vi "UHR-Fleezers Control (host) - 10.8MV_trial.vi"() -> ()   [LabVIEW 2010] (continued)
        n689 = local read "X RF Frequency Limits (MHz)"() -> (w3468:T16)
        n690 = local read "Y RF Frequency Limits (MHz)"() -> (w3465:T16)
        n691 = local read "BD 2 Frequency 1 (MHz)"() -> (w3470:dbl)
        n692 = Negate(x="Scan Range (nm)") -> (-x=w3434:dbl)
        n693 = Divide(x=w3434, y=w3456) -> (x/y=w3438:dbl)
        n694 = Select(t=w3468, s="Scan BD", f=w3465) -> (s? t:f=w3467:T16)
        n695 = Select(t=w3464, s="Scan BD", f=w3470) -> (s? t:f=w3469:dbl)
        n696 = Unbundle By Name(w3467) -> ("Maximum"=w3476:dbl, "Minimum"=w3475:dbl)
        n697 = Add(x=w3438, y=w3469) -> (x+y=w3473:dbl)
        n698 = Divide(x=w3434, y="Step Size (nm)") -> (x/y=w3453:dbl)
        n699 = Divide(x="Step Size (nm)", y=w3456) -> (x/y=w3462:dbl)
        n700 = Absolute Value(x=w3453) -> (abs(x)=w3437:dbl)
        n701 = Sign(1:w3434) -> (0:w3435:dbl)
        n702 = In Range and Coerce(upper limit=w3476, x=w3473, lower limit=w3475) -> (coerced(x)=w3472:dbl, In Range?=w3474:bool)
        n703 = To Unsigned Quad Integer(1:w3437) -> (0:w3452:u64)
        "Scan steps (AOD)" <- w3452
        n704 = call "IR AOM freq to word.vi"("Frequency In (MHz)"=w3462) -> ("Frequency Word Out (double)"=w3459:dbl)
        n705 = Multiply(x=w3435, y=w3459) -> (x*y=w3436:dbl)
        n706 = Subtract(x=w3473, y=w3472) -> (x-y=w3471:dbl)
        n707 = To Quad Integer(1:w3436) -> (0:w3458:i64)
        "Incr. int (AOD)" <- w3458
        n708 = Subtract(x=w3438, y=w3471) -> (x-y=w3457:dbl)
        "Scan Range (MHz)" <- w3457
        n709 = Select(t=w3438, s=w3474, f=w3457) -> (s? t:f=w3477:dbl)
        n710 = Multiply(x=w3457, y=w3456) -> (x*y=w3455:dbl)
        n711 = Decrement(x=w3452) -> (x-1=w3505:u64)
        n712 = Negate(x=w3455) -> (-x=w3451:dbl)
        n713 = local write "Scan Range (nm)"(w3451) -> ()
        n714 = Divide(x=w3477, y=w3505) -> (x/y=w3461:dbl)
        "Scan Increment (MHz)" <- w3461
        n715 = call "IR AOM freq to word.vi"("Frequency In (MHz)"=w3461) -> ("Frequency Word Out (double)"=w3460:dbl)
        n716 = Divide(x="Step Size (nm)", y="Scan Speed (nm/s)") -> (x/y=w3448:dbl)
        n717 = To Quad Integer(1:w3460) -> ()  [unwired: 1 out]
        n718 = local read "Number Interlace Sets"() -> (w3432:u8)
        n719 = local read "AI Count (ticks)"() -> (w3433:u32)
        n720 = local read "Total Counts (ticks)"() -> (w3431:u32)
        n721 = local read "# Samples/trap"() -> (w3463:u32)
        n722 = Multiply(x=w3433, y=w3432) -> (x*y=w3430:u32)
        n723 = Divide(x=w3431, y=w3430) -> (x/y=w3429:dbl)
        n724 = Select(t=w3464, s="Scan BD", f=w3470) -> (s? t:f=w3502:dbl)
        "Initial freq. (MHz)" <- w3502
        n725 = Add(x=w3477, y=w3502) -> (x+y=→"Final freq. (MHz)":dbl)
        n726 = Divide(x=w3431, y=40000000.0) -> (x/y=w3447:dbl)
        n727 = Divide(x=w3448, y=w3447) -> (x/y=w3446:dbl)
        n728 = To Unsigned Quad Integer(1:w3446) -> (0:w3421:u64)
        n729 = Quotient & Remainder(x=w3421, y=u64 2) -> (x-y*floor(x/y)=w3425:u64)  [unwired: 1 out]
        n730 = Equal?(x=w3425, y=u64 0) -> (x = y?=w3423:bool)
        n731 = Decrement(x=w3421) -> (x-1=w3422:u64)
        n732 = Select(t=w3421, s=w3423, f=w3422) -> (s? t:f=w3420:u64)
        "Cycles/step (AOD)" <- w3420
        n733 = xnode "Read/Write Control"("FPGA VI Reference In"=w3513, "error in"=w3512, "Scan steps"=w3452, "Number of scans"="Number of F/B Scans (AOD)", "Cycles per step"=w3420, "Scan freq.  increment"=w3458, "Scan BD"="Scan BD") -> ("error out"=w3511:errorcluster)  [unwired: 1 out]
        n734 = Multiply(x=w3452, y=w3420) -> (x*y=w3506:u64)
        n735 = Multiply(x=w3506, y=u64 2) -> (x*y=w3428:u64)
        n736 = Multiply(x=w3429, y=w3428) -> (x*y=w3427:dbl)
        "Data points/scan (f/b)" <- w3427
        n737 = Multiply(x=w3427, y="Number of F/B Scans (AOD)") -> (x*y=w3509:dbl)
        "Data points/scans" <- w3509
        n738 = Divide(x=w3509, y=w3463) -> (x/y=→"N sets should be saved":dbl)
        n739 = Multiply(x=w3506, y=w3447) -> (x*y=w3445:dbl)
        "Time/Scan (s) (AOD)" <- w3445
        n740 = Select(t=w3477, s="Scan BD", f=0.0) -> (s? t:f=w3503:dbl)
        n741 = Select(t=0.0, s="Scan BD", f=w3477) -> (s? t:f=w3499:dbl)
        n742 = local read "BD 2 Frequency 2 (MHz)"() -> (w3495:dbl)
        n743 = local read "BD 1 Frequency 2 (MHz)"() -> (w3498:dbl)
        n744 = Add(x=w3499, y=w3470) -> (x+y=w3496:dbl)
        n745 = Add(x=w3464, y=w3503) -> (x+y=w3497:dbl)
        n746 = Multiply(x=w3445, y=2.0) -> (x*y=w3444:dbl)
        n747 = Multiply(x=w3444, y="Number of F/B Scans (AOD)") -> (x*y=w3441:dbl)
        n748 = Divide(x=w3441, y=60.0) -> (x/y=→"Time to Finish All (min)":dbl)
        n749 = Add(x="Trap 2 Bead Size (nm)", y="Trap 1 Bead Size (nm)") -> (x+y=w3485:dbl)
        n750 = local read "Initial delta (MHz)"() -> (w3482:dbl)
        n751 = Divide(x=w3485, y=2.0) -> (x/y=w3479:dbl)
        n752 = Subtract(x=w3496, y=w3495) -> (x-y=w3493:dbl)
        n753 = Subtract(x=w3497, y=w3498) -> (x-y=w3494:dbl)
        n754 = Square(x=w3493) -> (x^2=w3492:dbl)
        n755 = Square(x=w3494) -> (x^2=w3491:dbl)
        n756 = Add(x=w3491, y=w3492) -> (x+y=w3490:dbl)
        n757 = Square Root(x=w3490) -> (sqrt(x)=w3489:dbl)
        "Final delta (MHz)" <- w3489
        n758 = Multiply(x=w3481, y=w3489) -> (x*y=w3488:dbl)
        n759 = Multiply(x=w3482, y=w3481) -> (x*y=w3480:dbl)
        n760 = Subtract(x=w3480, y=w3479) -> (x-y=→"Initial sep (nm)":dbl)
        n761 = Subtract(x=w3488, y=w3479) -> (x-y=→"Final sep (nm)":dbl)
      }
      event "Raster Scanning...": Value Change {
        n762 = event-data() -> ("NewVal"=w3650:bool)  [unwired: 6 out]
        n763 = case shown="True" w3650 {
          frame False {
          }
          frame True {
            n764 = property on="BD 1 Frequency 1 (MHz)" class="DigNum (strict)"("Val(Sgnl)"=65.0 ("Value (Signaling)")) -> ()  [unwired: 2 in, 2 out]
          }
        }
      }
      event "Freq or Amp switch first", "Swap F1 and F2", "Freq switch delay", "Amp switch delay": Value Change {
        n765 = event-data() -> ()  [unwired: 7 out]
        n766 = local read "Freq or Amp switch first"() -> (w3652:bool)
        n767 = local read "Amp switch delay"() -> (w3653:u16)
        n768 = local read "Freq switch delay"() -> (w3655:u16)
        n769 = local read "Swap F1 and F2"() -> (w3654:bool)
        n770 = xnode "Read/Write Control"("FPGA VI Reference In"=w3658, "error in"=w3657, "Freq switch delay"=w3655, "Swap F1 and F2"=w3654, "Amp switch delay"=w3653, "Freq or Amp switch first"=w3652) -> ("error out"=w3656:errorcluster)  [unwired: 1 out]
      }
      event "Scan steps (MCL)", "Number of scans (MCL)", "Scan Range (V)\n(of steps)", "2D or 1D Scan", "N APD Samp/step", "Fast Scan Dir", "Continuous MCL Scanning", "Scan lines (y)": Value Change {
        w3759 = 32767.0 ("y")
        n771 = event-data() -> ()  [unwired: 7 out]
        n772 = Select(t="Scan lines (y)", s="2D or 1D Scan", f="Number of scans (MCL)") -> (s? t:f=w3764:u64)
        n773 = Decrement(x="Scan steps (MCL)") -> (x-1=w3780:u64)
        n774 = Divide(x="Scan Range (V)\n(of steps)", y=w3780) -> (x/y=w3779:dbl)
        "Desired Scan Incr (V)" <- w3779
        n775 = local read "APD Integration Time (s)"() -> (w3772:dbl)
        n776 = Multiply(x=w3779, y=w3759) -> (x*y=w3788:dbl)
        n777 = Divide(x=w3788, y=10.0) -> (x/y=w3778:dbl)
        "Desired incr (int)" <- w3778
        n778 = local read "Update Count (MCL)"() -> (w3784:u32)
        n779 = Round Toward -Infinity(1:w3778) -> (0:w3787:dbl)
        n780 = To Word Integer(number=w3787) -> (16bit integer=w3762:i16)
        "Actual Incr. int (MCL)" <- w3762
        n781 = Multiply(x=w3772, y=40000000.0) -> (x*y=w3785:dbl)
        n782 = Divide(x=w3785, y=w3784) -> (x/y=w3783:dbl)
        n783 = Multiply(x=i16 10, y=w3762) -> (x*y=w3760:i16)
        n784 = Multiply(x="N APD Samp/step", y=w3783) -> (x*y=w3782:dbl)
        "Cycles/step (MCL)" <- w3782
        n785 = Divide(x=w3760, y=w3759) -> (x/y=→"Actual MCL Inc (V)":dbl)
        n786 = Multiply(x="N APD Samp/step", y="Scan steps (MCL)") -> (x*y=w3774:dbl)
        n787 = local read "APD Samples/FIFO Acq."() -> (w3771:dbl)
        n788 = Multiply(x=w3774, y=u64 2) -> (x*y=w3773:dbl)
        "Data points/scan (f+b)" <- w3773
        n789 = Multiply(x=w3773, y=w3764) -> (x*y=w3791:dbl)
        "Data points/scans (MCL)" <- w3791
        n790 = Multiply(x=w3772, y=w3773) -> (x*y=w3765:dbl)
        "Time/f+b scan (s) (MCL)" <- w3765
        n791 = Divide(x=w3791, y=w3771) -> (x/y=→"N sets should be saved (MCL)":dbl)
        n792 = Multiply(x=w3765, y=w3764) -> (x*y=→"Total Time (s)":dbl)
        n793 = Not(x="Fast Scan Dir") -> (.not. x?=w3769:bool)
        n794 = xnode "Read/Write Control"("FPGA VI Reference In"=w3795, "error in"=w3794, "Scan steps (MCL)"="Scan steps (MCL)", "Number of scans (MCL)"=w3764, "Cycles per step (MCL)"=w3782, "Scan freq.  increment (MCL)"=w3762, "1D or 2D Scan?"="2D or 1D Scan", "MCL Scan Axis"=w3769, "Cont. Scan (MCL)"="Continuous MCL Scanning") -> ("error out"=w3793:errorcluster)  [unwired: 1 out]
      }
      event "Read Cal": Value Change {
        w3969 = 1000.0 ("y")
        n795 = event-data() -> ()  [unwired: 7 out]
        n796 = local read "Save file name"() -> (w3994:path)
        n797 = local write "Read Cal"(FALSE ("Read Cal")) -> ()
        n798 = Strip Path(path=w3994) -> (stripped path=w3993:path)  [unwired: 1 out]
        n799 = Path To String(path=w3993) -> (string=w3992:string)
        n800 = Concatenate Strings(w3992, "\\current.cal" ("string")) -> (w3990:string)
        n801 = String To Path(string=w3990) -> (path=w3989:path)
        n802 = Open/Create/Replace File(file path (use dialog)=w3989, operation (0:open)=T25."open", access (0:read/write)=enum16{"read/write", "read-only", "write-only"}."read-only") -> (refnum out=w3997:refnum<file>, error out=w3983:errorcluster)  [unwired: 1 in, 3 out]
        n803 = Deny Access(4:w3983, 7:w3997) -> (0:w3982:errorcluster, 3:w3988:refnum<file>)  [unwired: 1 out]
        n804 = Read from Binary File(5:0.0, 8:w3982, 9:T31."big-endian, network order" ("byte order (0:big-endian, network order)"), 10:-1 ("count (1)"), 11:w3988) -> (0:w3981:errorcluster, 2:w3979:dbl[], 3:w3984:refnum<file>)  [unwired: 2 out]
        n805 = Array To Cluster(array=w3979) -> (cluster=w3978:T33)
        n806 = Unbundle(w3978) -> ("[0]"=w3977:dbl, "[1]"=w3976:dbl, "[2]"=w3975:dbl, "[3]"=w3974:dbl, "[4]"=w3973:dbl, "[5]"=w3972:dbl)
        n807 = Close File(refnum=w3984, error in=w3981) -> (error out=→"Read cal error":errorcluster)  [unwired: 1 out]
        n808 = Multiply(x=w3972, y=w3969) -> (x*y=w3970:dbl)
        n809 = local write "T2 kappa_x (pN/nm)"(w3974) -> ()
        n810 = local write "T1 kappa_x (pN/nm)"(w3975) -> ()
        n811 = local write "T1 alpha_x (nm/V)"(w3977) -> ()
        n812 = local write "T2 alpha_x (nm/V)"(w3976) -> ()
        n813 = Multiply(x=w3973, y=w3969) -> (x*y=w3971:dbl)
        n814 = local write "T1 offset_x (mV)"(w3971) -> ()
        n815 = local write "T2 offset_x (mV)"(w3970) -> ()
      }
      event "Abort MCL Scan": Value Change {
        n816 = event-data() -> ()  [unwired: 7 out]
        n817 = local write "MCL Scanning"(FALSE ("MCL Scanning")) -> ()
        n818 = xnode "Read/Write Control"("FPGA VI Reference In"=w4002, "error in"=w4001, "Abort scan (MCL)"="Abort MCL Scan") -> ("error out"=w4000:errorcluster)  [unwired: 1 out]
      }
      event "Update Count (MCL)": Value Change {
        n819 = event-data() -> ()  [unwired: 7 out]
        n820 = xnode "Read/Write Control"("FPGA VI Reference In"=w4044, "error in"=w4043, "MCL count"="Update Count (MCL)") -> ("error out"=w4042:errorcluster)  [unwired: 1 out]
      }
      event "Phase adjust (MCL)", "+ phase (MCL)", "- phase (MCL)": Value Change {
        n821 = event-data() -> ()  [unwired: 7 out]
        n822 = Negate(x="Phase adjust (MCL)") -> (-x=w4090:i16)
        n823 = Select(t=w4090, s="- phase (MCL)", f="Phase adjust (MCL)") -> (s? t:f=w4088:i16)
        n824 = Or(x="- phase (MCL)", y="+ phase (MCL)") -> (x .or. y?=w4083:bool)
        n825 = xnode "Read/Write Control"("FPGA VI Reference In"=w4092, "error in"=w4091, "Phase count adjustment (MCL)"=w4088) -> ("FPGA VI Reference Out"=w4084:T19, "error out"=w4085:errorcluster)
        n826 = xnode "Read/Write Control"("FPGA VI Reference In"=w4084, "error in"=w4085, "+ phase (MCL)"=w4083) -> ("error out"=w4082:errorcluster)  [unwired: 1 out]
      }
      event "Abort AOD Scan": Value Change {
        n827 = event-data() -> ()  [unwired: 7 out]
        n828 = xnode "Read/Write Control"("FPGA VI Reference In"=w4171, "error in"=w4170, "Abort scan"="Abort AOD Scan") -> ("error out"=w4169:errorcluster)  [unwired: 1 out]
      }
      event "Continuous AOD Scanning": Value Change {
        n829 = event-data() -> ()  [unwired: 7 out]
        n830 = xnode "Read/Write Control"("FPGA VI Reference In"=w4213, "error in"=w4212, "Cont. Scan"="Continuous AOD Scanning") -> ("error out"=w4211:errorcluster)  [unwired: 1 out]
      }
      event "Index": Value Change {
        n831 = event-data() -> ()  [unwired: 7 out]
        n832 = call "Create new save file.vi"("Insert"="", "Ext"=".dat" ("string"), "Index In"="Index") -> ("Path Out"=→"Save file name":path, "Index Out"=w4252:dbl)
        "Save index" <- w4252
        n833 = local write "Index"(w4252) -> ()
      }
      event "AO1", "AO2": Value Change {
        w4267 = 10.0 ("y")
        w4266 = 32767.0 ("y")
        n834 = event-data() -> ()  [unwired: 7 out]
        n835 = local read "AO2"() -> (w4265:dbl)
        n836 = local read "AO1"() -> (w4262:dbl)
        n837 = Multiply(x=w4262, y=w4266) -> (x*y=w4261:dbl)
        n838 = Multiply(x=w4265, y=w4266) -> (x*y=w4264:dbl)
        n839 = Divide(x=w4261, y=w4267) -> (x/y=w4260:dbl)
        n840 = Divide(x=w4264, y=w4267) -> (x/y=w4263:dbl)
        n841 = To Word Integer(number=w4260) -> (16bit integer=w4268:i16)
        n842 = To Word Integer(number=w4263) -> (16bit integer=w4269:i16)
        n843 = xnode "Read/Write Control"("FPGA VI Reference In"=w4259, "error in"=w4258, "AO1"=w4268, "AO2"=w4269) -> ("error out"=w4257:errorcluster)  [unwired: 1 out]
      }
      event "Inject Bottom": Value Change {
        n844 = event-data() -> ()  [unwired: 7 out]
        n845 = disable-structure shown="Enabled" {
          disable-tunnel: "Inject Bottom" -> [w4328 w4368]
          frame Disabled {
            n846 = local read "Chemyx Syringe Pump Serial Port"() -> (w4329:refnum<visa-resource-name>)
            n847 = local read "Pump write delay (ms)"() -> (w4330:dbl)
            n848 = case shown="True" w4328 {
              tunnel: w4330 -> [w4336 w4350]
              tunnel: w4329 -> [w4333 w4349]
              frame False {
                n849 = flat-sequence {
                  tunnel: w4333 -> [w4337]
                  tunnel: [w4337] -> w4334
                  tunnel: w4336 -> [_]
                  tunnel: [w4340] -> w4335
                  tunnel: w4334 -> [w4340]
                  tunnel: w4335 -> [w4341]
                  tunnel: [w4341] -> w4331
                  tunnel: [w4343] -> w4332
                  tunnel: w4331 -> [w4343]
                  tunnel: w4332 -> [w4345]
                  frame #0 {
                    n850 = call "Write to pump.vi"("string"="enter pump1", "VISA resource name"=w4337) -> ()  [unwired: 1 out]
                  }
                  frame #1 {
                    n851 = Wait (ms)(milliseconds to wait="Pump pause delay (ms)") -> ()  [unwired: 1 out]
                  }
                  frame #2 {
                    n852 = call "Write to pump.vi"("string"="stop", "VISA resource name"=w4341) -> ()  [unwired: 1 out]
                  }
                  frame #3 {
                    n853 = Wait (ms)(milliseconds to wait=u32 500) -> ()  [unwired: 1 out]
                  }
                  frame #4 {
                    n854 = call "Write to pump.vi"("string"="stop", "VISA resource name"=w4345) -> ()  [unwired: 1 out]
                  }
                }
              }
              frame True {
                n855 = flat-sequence {
                  tunnel: w4349 -> [w4359]
                  tunnel: w4350 -> [w4354]
                  tunnel: w4350 -> [w4361]
                  tunnel: w4349 -> [w4362]
                  tunnel: [w4362] -> w4347
                  tunnel: [w4364] -> w4348
                  tunnel: w4347 -> [w4364]
                  tunnel: w4348 -> [w4366]
                  frame #0 {
                    n856 = local read "All Pump Parameters"() -> (w4353:T5)
                    n857 = Unbundle By Name(w4353) -> ("Pump 1"=w4360:T34)
                    n858 = call "Set pump parameters.vi"("Pump write delay (ms)"=w4354, "Volume (uL)"="Ch 2 Inject Volume (uL)", "Rate (uL/h)"="Ch 1 Inject Rate (ul/h)", "Units"=4.0, "Pump #"=1.0, "Pump Parameters In"=w4360, "VISA resource name"=w4359) -> ("Pump Parameters Out"=w4352:T34)  [unwired: 3 in]
                    n859 = Bundle By Name(cluster=w4353, "Pump 1"=w4352) -> (w4351:T5)
                    n860 = local write "All Pump Parameters"(w4351) -> ()
                  }
                  frame #1 {
                    n861 = Wait (ms)(milliseconds to wait=w4361) -> ()  [unwired: 1 out]
                  }
                  frame #2 {
                    n862 = call "Write to pump.vi"("string"="start", "VISA resource name"=w4362) -> ()  [unwired: 1 out]
                  }
                  frame #3 {
                    n863 = Wait (ms)(milliseconds to wait=u32 500) -> ()  [unwired: 1 out]
                  }
                  frame #4 {
                    n864 = call "Write to pump.vi"("string"="start", "VISA resource name"=w4366) -> ()  [unwired: 1 out]
                  }
                }
              }
            }
          }
          frame Enabled {
            n865 = call "hamilton_controller.vi"("Open?"=w4368, "valve"=enum16{"A", "B", "C", "D", "ALL"}."B", "action"=T22."MOVE VALVE") -> ()  [unwired: 8 in, 1 out]
          }
        }
      }
      event "Inject Top": Value Change {
        n866 = event-data() -> ()  [unwired: 7 out]
        n867 = disable-structure shown="Disabled" {
          disable-tunnel: "Inject Top" -> [_ w4412]
          frame Disabled {
            n868 = local read "Pump write delay (ms)"() -> (w4373:dbl)
            n869 = case shown="False" w4374 {
              tunnel: w4373 -> [w4380 w4394]
              tunnel: "Chemyx Syringe Pump Serial Port" -> [w4377 w4393]
              frame False {
                n870 = flat-sequence {
                  tunnel: w4377 -> [w4381]
                  tunnel: [w4381] -> w4378
                  tunnel: w4380 -> [_]
                  tunnel: [w4384] -> w4379
                  tunnel: w4378 -> [w4384]
                  tunnel: w4379 -> [w4385]
                  tunnel: [w4385] -> w4375
                  tunnel: [w4387] -> w4376
                  tunnel: w4375 -> [w4387]
                  tunnel: w4376 -> [w4389]
                  frame #0 {
                    n871 = call "Write to pump.vi"("string"="enter pump3", "VISA resource name"=w4381) -> ()  [unwired: 1 out]
                  }
                  frame #1 {
                    n872 = local read "Pump pause delay (ms)"() -> (w4383:u32)
                    n873 = Wait (ms)(milliseconds to wait=w4383) -> ()  [unwired: 1 out]
                  }
                  frame #2 {
                    n874 = call "Write to pump.vi"("string"="stop", "VISA resource name"=w4385) -> ()  [unwired: 1 out]
                  }
                  frame #3 {
                    n875 = Wait (ms)(milliseconds to wait=u32 0) -> ()  [unwired: 1 out]
                  }
                  frame #4 {
                    n876 = call "Write to pump.vi"("string"="stop", "VISA resource name"=w4389) -> ()  [unwired: 1 out]
                  }
                }
              }
              frame True {
                n877 = flat-sequence {
                  tunnel: w4393 -> [w4403]
                  tunnel: w4394 -> [w4398]
                  tunnel: w4394 -> [w4405]
                  tunnel: w4393 -> [w4406]
                  tunnel: [w4406] -> w4391
                  tunnel: [w4409] -> w4392
                  tunnel: w4391 -> [w4409]
                  tunnel: w4392 -> [w4410]
                  frame #0 {
                    n878 = local read "All Pump Parameters"() -> (w4397:T5)
                    n879 = Unbundle By Name(w4397) -> ("Pump 3"=w4404:T34)
                    n880 = call "Set pump parameters.vi"("Pump write delay (ms)"=w4398, "Volume (uL)"="Ch 3 Inject Volume (uL)", "Rate (uL/h)"="Ch 3 Inject Rate (ul/h)", "Units"=4.0, "Pump #"=3.0, "Pump Parameters In"=w4404, "VISA resource name"=w4403) -> ("Pump Parameters Out"=w4396:T34)  [unwired: 3 in]
                    n881 = Bundle By Name(cluster=w4397, "Pump 3"=w4396) -> (w4395:T5)
                    n882 = local write "All Pump Parameters"(w4395) -> ()
                  }
                  frame #1 {
                    n883 = Wait (ms)(milliseconds to wait=w4405) -> ()  [unwired: 1 out]
                  }
                  frame #2 {
                    n884 = call "Write to pump.vi"("string"="start", "VISA resource name"=w4406) -> ()  [unwired: 1 out]
                  }
                  frame #3 {
                    n885 = Wait (ms)(milliseconds to wait=u32 500) -> ()  [unwired: 1 out]
                  }
                  frame #4 {
                    n886 = call "Write to pump.vi"("string"="start", "VISA resource name"=w4410) -> ()  [unwired: 1 out]
                  }
                }
              }
            }
          }
          frame Enabled {
            n887 = call "hamilton_controller.vi"("Open?"=w4412, "valve"=enum16{"A", "B", "C", "D", "ALL"}."A", "action"=T22."MOVE VALVE") -> ()  [unwired: 8 in, 1 out]
          }
        }
      }
      event "Inject Valve B": Value Change {
        n888 = event-data() -> ()  [unwired: 7 out]
        n889 = disable-structure shown="Enabled" {
          disable-tunnel: "Inject Valve B" -> [w4416 w4436]
          frame Disabled {
            n890 = local read "Pump write delay (ms)"() -> (w4418:dbl)
            n891 = flat-sequence {
              tunnel: w4417 -> [w4431]
              tunnel: w4418 -> [w4427]
              tunnel: w4416 -> [_]
              tunnel: w4418 -> [w4433]
              tunnel: w4417 -> [w4434]
              frame #0 {
                n892 = local read "All Pump Parameters"() -> (w4426:T5)
                n893 = Multiply(x=60.0, y="Flush Center Ch Rate (ul/m)") -> (x*y=w4423:dbl)
                n894 = Unbundle By Name(w4426) -> ("Pump 2"=w4432:T34)
                n895 = call "Set pump parameters.vi"("Pump write delay (ms)"=w4427, "Volume (uL)"="Flush Center Ch Volume (uL)", "Rate (uL/h)"=w4423, "Units"=3.0, "Pump #"=2.0, "Pump Parameters In"=w4432, "VISA resource name"=w4431) -> ("Pump Parameters Out"=w4425:T34)  [unwired: 3 in]
                n896 = Bundle By Name(cluster=w4426, "Pump 2"=w4425) -> (w4424:T5)
                n897 = local write "All Pump Parameters"(w4424) -> ()
                n898 = Add(x="Flush Center Ch Volume (uL)", y="Total Volume\nFlushed (uL)") -> (x+y=w4420:dbl)
                n899 = local write "Total Volume\nFlushed (uL)"(w4420) -> ()
              }
              frame #1 {
                n900 = Wait (ms)(milliseconds to wait=w4433) -> ()  [unwired: 1 out]
              }
              frame #2 {
                n901 = call "Write to pump.vi"("string"="start", "VISA resource name"=w4434) -> ()  [unwired: 1 out]
              }
            }
            n902 = local read "Chemyx Syringe Pump Serial Port"() -> (w4417:refnum<visa-resource-name>)
          }
          frame Enabled {
            n903 = call "hamilton_controller.vi"("Open?"=w4436, "valve"=enum16{"A", "B", "C", "D", "ALL"}."B", "action"=T22."MOVE VALVE") -> ()  [unwired: 8 in, 1 out]
          }
        }
      }
      event "Sample Channel Flow": Value Change {
        n904 = event-data() -> ()  [unwired: 7 out]
        n905 = call "hamilton_controller.vi"("Open?"="Sample Channel Flow", "valve"=enum16{"A", "B", "C", "D", "ALL"}."C", "action"=T22."MOVE VALVE") -> ()  [unwired: 8 in, 1 out]
      }
      event "Flip Green Filter": Value Change {
        n906 = event-data() -> ()  [unwired: 7 out]
        n907 = Not(x="Flip Green Filter") -> (.not. x?=w4442:bool)
        n908 = local write "Flip Green Filter"(w4442) -> ()
        n909 = flat-sequence {
          tunnel: w4450 -> [w4455]
          tunnel: w4449 -> [w4454]
          tunnel: [w4452] -> w4447
          tunnel: [w4451] -> w4446
          tunnel: [w4495] -> w4445
          tunnel: w4447 -> [w4495]
          tunnel: [w4494] -> w4444
          tunnel: w4446 -> [w4494]
          tunnel: w4445 -> [w4499]
          tunnel: w4444 -> [w4498]
          tunnel: [w4497] -> w4448
          frame #0 {
            n910 = xnode "Read/Write Control"("FPGA VI Reference In"=w4455, "error in"=w4454, "Green Filter Flipper"=TRUE) -> ("FPGA VI Reference Out"=w4452:T19, "error out"=w4451:errorcluster)
          }
          frame #1 {
            n911 = Wait (ms)(milliseconds to wait=u32 100) -> ()  [unwired: 1 out]
          }
          frame #2 {
            n912 = xnode "Read/Write Control"("FPGA VI Reference In"=w4499, "error in"=w4498, "Green Filter Flipper"=FALSE) -> ("error out"=w4497:errorcluster)  [unwired: 1 out]
          }
        }
      }
      event "Pump 1 contents", "Pump 3 contents": Value Change {
        n913 = event-data() -> ()  [unwired: 7 out]
        n914 = local read "Pump 1 contents"() -> (→"Pump 1 cont disp":string)
        n915 = local read "Pump 3 contents"() -> (→"Pump 3 cont disp":string)
      }
      event "Reset Trap Pos. FB": Value Change {
        n916 = event-data() -> ()  [unwired: 7 out]
        n917 = xnode "Read/Write Control"("FPGA VI Reference In"=w4543, "error in"=w4542, "Trap Pos. FB Reset"="Reset Trap Pos. FB") -> ()  [unwired: 2 out]
      }
      event "Trap Pos. FB ON": Value Change {
        n918 = event-data() -> ()  [unwired: 7 out]
        n919 = xnode "Read/Write Control"("FPGA VI Reference In"=w4584, "error in"=w4583, "Force feedback"="Trap Pos. FB ON") -> ()  [unwired: 2 out]
      }
      event "Trap Pos. FB Range", "Trap Pos. FB Gains", "Trap Pos. FB Mult Factor", "Trap Pos. FB Offset Factor", "Trap Pos FB Negate Action", "Trap Pos FB Monitor\nT1 or T2": Value Change {
        n920 = event-data() -> ()  [unwired: 7 out]
        n921 = xnode "Read/Write Control"("FPGA VI Reference In"=w4631, "error in"=w4630, "Trap Pos. FB Range"="Trap Pos. FB Range", "Trap Pos. FB Gains"="Trap Pos. FB Gains", "Trap Pos. FB Mult Factor"="Trap Pos. FB Mult Factor", "Trap Pos. FB Offset Factor"="Trap Pos. FB Offset Factor", "Trap Pos FB Negate Action"="Trap Pos FB Negate Action", "Trap Pos FB Monitor T1 or T2"="Trap Pos FB Monitor\nT1 or T2", "AI1 X Scale"="Trap Pos. AI1 X Pre-scale") -> ()  [unwired: 2 out]
      }
      event "Trap Pos FB SP": Value Change {
        n922 = event-data() -> ()  [unwired: 7 out]
        n923 = xnode "Read/Write Control"("FPGA VI Reference In"=w4819, "error in"=w4818, "Trap Pos. FB SP"="Trap Pos FB SP") -> ()  [unwired: 2 out]
      }
      event "Set SP to Reading": Value Change {
        n924 = event-data() -> ()  [unwired: 7 out]
        n925 = local read "Trap Pos FB Monitor\nT1 or T2"() -> (w4872:bool)
        n926 = local read "Trap X AI1 (DMA)"() -> (w4875:T13)
        n927 = local read "Trap X (AI1)"() -> (w4878:T10)
        n928 = Unbundle By Name(w4878) -> ("Trap 1"=w4877:fxp<+/-,16,1>, "Trap 2"=w4876:fxp<+/-,16,1>)
        n929 = Unbundle By Name(w4875) -> ("Set 1"=w4874:fxp<+/-,16,1>, "Set 2"=w4873:fxp<+/-,16,1>)
        n930 = Select(t=w4877, s=w4872, f=w4876) -> (s? t:f=w4871:fxp<+/-,16,1>)
        n931 = Select(t=w4874, s=w4872, f=w4873) -> (s? t:f=w4870:fxp<+/-,16,1>)
        n932 = Not(x="Set SP Using...") -> (.not. x?=w4865:bool)
        n933 = Select(t=w4871, s=w4865, f=w4870) -> (s? t:f=w4866:fxp<+/-,16,1>)
        n934 = xnode "Read/Write Control"("FPGA VI Reference In"=w4868, "error in"=w4867, "Trap Pos. FB SP"=w4866) -> ()  [unwired: 2 out]
        n935 = local write "Trap Pos FB SP"(w4866) -> ()
      }
      event "Trap Pos. FB Out Scale 2^n": Value Change {
        n936 = event-data() -> ()  [unwired: 7 out]
        n937 = Scale By Power Of 2(n="Trap Pos. FB Out Scale 2^n", x=ext 1.0) -> (x*2^n=w4925:ext)
        n938 = property on="Trap Pos. FB Mult Factor" class="DigNum (strict)"("Val(Sgnl)"=w4925) -> ()  [unwired: 2 in, 2 out]
      }
      event "Trap Pos FB Int Count": Value Change {
        n939 = event-data() -> ()  [unwired: 7 out]
        n940 = xnode "Read/Write Control"("FPGA VI Reference In"=w4930, "error in"=w4929, "Trap Pos FB Int Count"="Trap Pos FB Int Count") -> ()  [unwired: 2 out]
      }
    }
    "error out 2" <- w1255
    n941 = node-c288() -> ()  [unwired: 1 in, 1 out]
  }
  n942 = timed-loop "Run Scripts, including: stage motion" {
    timing: w69 -> [_]
    timing-out: [_] -> w68
    tunnel: w24 -> [_]
    stop <- w4969 stop-if-true
    n943 = node-c288() -> ()  [unwired: 1 in, 1 out]
    n944 = event shown="[2] \"Cal/Data Acq. Spot\": Value Change" {
      selector: _ -> [_ _ _ _ _ _ _ _ _ _ _ _]
      dyn-events: _ -> [_ _ _ _ _ _ _ _ _ _ _ _]
      timeout: 50 -> [_ _ _ _ _ _ _ _ _ _ _ _]
      tunnel: ["Move Cap. 1 (DNA Top)" _ "Cal/Data Acq. Spot" "Dump Beads" "Dip for Protein" _ "Got ADig bead" "Got DNA bead" "Take Stepping Data" _ "Take Detection Laser\nImage" _] -> _
      tunnel: [_ _ _ _ _ _ _ _ _ _ _ w5173] -> w4969
      event "Move Cap. 1 (DNA Top)": Value Change {
        n945 = event-data() -> ()  [unwired: 1 in, 5 out]
        n946 = local write "Move Cap. 1 (DNA Top)"(FALSE ("Move Cap. 1 (DNA Right)")) -> ()
        n947 = flat-sequence {
          tunnel: "Cap 1 Samp Flow ON" -> [w4975]
          frame #0 {
            n948 = local write "Stage Moving"(FALSE ("Stage Moving")) -> ()
            n949 = case "stop flow" shown="True" w4975 {
              frame False {
              }
              frame True {
                n950 = call "hamilton_controller.vi"("Open?"=FALSE, "valve"=enum16{"A", "B", "C", "D", "ALL"}."C", "action"=T22."MOVE VALVE") -> ()  [unwired: 8 in, 1 out]
              }
            }
            n951 = case shown="True" TRUE {
              tunnel: "Cap 1 T ON" -> [w4984 w4985]
              frame False {
                n952 = property on="Trap 1 (ON/OFF)" class="Bool (strict)"("Val(Sgnl)"=w4984) -> ()  [unwired: 2 in, 2 out]
              }
              frame True {
                n953 = property on="Trap 2 (ON/OFF)" class="Bool (strict)"("Val(Sgnl)"=w4985) -> ()  [unwired: 2 in, 2 out]
              }
            }
            n954 = call <vilib>:"Beep.vi"() -> ()  [unwired: 3 in, 9 out]
            n955 = case shown="True" "Cap 1 Flow ON" {
              frame False {
              }
              frame True {
                n956 = property on="Inject Top" class="Bool (strict)"("Val(Sgnl)"=TRUE ("Value (Signaling)")) -> ()  [unwired: 2 in, 2 out]
              }
            }
          }
        }
      }
      event Timeout {
        n957 = event-data() -> ()  [unwired: 1 in, 2 out]
      }
      event "Cal/Data Acq. Spot": Value Change {
        # "wait for calibration file\nto be written"
        # "signal save cal true\nthis tells the data \nacquisition loop to\nstart sending the data\nto a calibration file"
        # "separate traps to\nthe desired trap delta"
        # "move stage to data acquisition spot"
        # "CHANGE FISH FOR TETHER BACK\nTO TRUE VALUE HERE."
        n958 = event-data() -> ()  [unwired: 1 in, 5 out]
        n959 = local write "Cal/Data Acq. Spot"(FALSE ("Cal/Data Acq. Spot")) -> ()
        n960 = flat-sequence {
          tunnel: ["Cal @ (MHz)"] -> w4986
          tunnel: w4986 -> [w4996]
          tunnel: w4986 -> [w5017]
          frame #0 {
            n961 = property on="Trap Delta (MHz)" class="DigNum (strict)"("Val(Sgnl)"="Cal @ (MHz)") -> ()  [unwired: 2 in, 2 out]
            n962 = call <vilib>:"Beep.vi"() -> ()  [unwired: 3 in, 9 out]
          }
          frame #1 {
            n963 = Wait (ms)(milliseconds to wait=u32 100) -> ()  [unwired: 1 out]
          }
          frame #2 {
            n964 = property on="Save Calibration" class="Bool (strict)"("Val(Sgnl)"=TRUE ("Value (Signaling)")) -> ()  [unwired: 2 in, 2 out]
          }
          frame #3 {
            n965 = Wait (ms)(milliseconds to wait=u32 4000) -> ()  [unwired: 1 out]
          }
          frame #4 {
            n966 = while {
              stop <- w4993 stop-if-true
              n967 = local read "Saving..."() -> (w4994:bool)
              n968 = Wait (ms)(milliseconds to wait=u32 100) -> ()  [unwired: 1 out]
              n969 = Not(x=w4994) -> (.not. x?=w4993:bool)
            }
          }
          frame #5 {
            n970 = case shown="True" "W/ Offset 1" {
              tunnel: w4996 -> [_ w4998]
              frame False {
              }
              frame True {
                n971 = stacked-sequence {
                  tunnel: w4998 -> [_ _ _ _ _ _ _ w5015]
                  frame #0 {
                    n972 = Replace Array Subset(array=u32[] [0] ("Index Values"), new element="Offset 1 Set", index=0) -> (w4999:u32[])
                    n973 = property on="Saved AOD Raster Scan Parameter Sets" class="Arr (strict)"("Index Values"=w4999) -> ()  [unwired: 2 in, 2 out]
                    n974 = property on="Trap Delta (MHz)" class="DigNum (strict)"("Val(Sgnl)"="Offset 1 Start (MHz)") -> ()  [unwired: 2 in, 2 out]
                  }
                  frame #1 {
                    n975 = Wait (ms)(milliseconds to wait=u32 200) -> ()  [unwired: 1 out]
                  }
                  frame #2 {
                    n976 = property on="Load parameters" class="Bool (strict)"("Val(Sgnl)"=TRUE ("Value (Signaling)")) -> ()  [unwired: 2 in, 2 out]
                  }
                  frame #3 {
                    n977 = Wait (ms)(milliseconds to wait=u32 200) -> ()  [unwired: 1 out]
                  }
                  frame #4 {
                    n978 = property on="Trap Raster Scan" class="Bool (strict)"("Val(Sgnl)"=TRUE ("Value (Signaling)")) -> ()  [unwired: 2 in, 2 out]
                  }
                  frame #5 {
                    n979 = Wait (ms)(milliseconds to wait=u32 2000) -> ()  [unwired: 1 out]
                  }
                  frame #6 {
                    n980 = while {
                      stop <- w5012 stop-if-true
                      n981 = local read "Raster Scanning..."() -> (w5014:bool)
                      n982 = local read "Saving..."() -> (w5010:bool)
                      n983 = Wait (ms)(milliseconds to wait=u32 100) -> ()  [unwired: 1 out]
                      n984 = Not(x=w5010) -> (.not. x?=w5009:bool)
                      n985 = Not(x=w5014) -> (.not. x?=w5011:bool)
                      n986 = And(x=w5011, y=w5009) -> (x .and. y?=w5012:bool)
                    }
                  }
                  frame #7 {
                    n987 = property on="Trap Delta (MHz)" class="DigNum (strict)"("Val(Sgnl)"=w5015) -> ()  [unwired: 2 in, 2 out]
                  }
                }
              }
            }
          }
          frame #6 {
            n988 = local read "Save ave N"() -> (w5016:dbl)
            n989 = case shown="True" "W/ Offset 2" {
              tunnel: w5017 -> [_ w5023]
              tunnel: w5016 -> [_ w5022]
              frame False {
                n990 = Multiply(x="Cal read wait (s)", y=u32 1000 ("milliseconds to wait")) -> (x*y=w5020:u32)
                n991 = Wait (ms)(milliseconds to wait=w5020) -> ()  [unwired: 1 out]
              }
              frame True {
                n992 = stacked-sequence {
                  tunnel: w5023 -> [_ _ _ _ _ _ _ _ _ w5044 _ _]
                  tunnel: w5022 -> [_ _ _ _ _ _ _ _ _ w5042 _ _]
                  frame #0 {
                    n993 = property on="Save ave N" class="DigNum (strict)"("Val(Sgnl)"=1.0 ("Value (Signaling)")) -> ()  [unwired: 2 in, 2 out]
                  }
                  frame #1 {
                    n994 = Wait (ms)(milliseconds to wait=u32 500) -> ()  [unwired: 1 out]
                  }
                  frame #2 {
                    n995 = property on="Trap Delta (MHz)" class="DigNum (strict)"("Val(Sgnl)"="Offset 2 Start (MHz)") -> ()  [unwired: 2 in, 2 out]
                    n996 = Replace Array Subset(array=u32[] [0] ("Index Values"), new element="Offset 2 Set", index=0) -> (w5028:u32[])
                    n997 = property on="Saved AOD Raster Scan Parameter Sets" class="Arr (strict)"("Index Values"=w5028) -> ()  [unwired: 2 in, 2 out]
                  }
                  frame #3 {
                    n998 = Wait (ms)(milliseconds to wait=u32 500) -> ()  [unwired: 1 out]
                  }
                  frame #4 {
                    n999 = property on="Load parameters" class="Bool (strict)"("Val(Sgnl)"=TRUE ("Value (Signaling)")) -> ()  [unwired: 2 in, 2 out]
                  }
                  frame #5 {
                    n1000 = Wait (ms)(milliseconds to wait=u32 500) -> ()  [unwired: 1 out]
                  }
                  frame #6 {
                    n1001 = property on="Trap Raster Scan" class="Bool (strict)"("Val(Sgnl)"=TRUE ("Value (Signaling)")) -> ()  [unwired: 2 in, 2 out]
                  }
                  frame #7 {
                    n1002 = Wait (ms)(milliseconds to wait=u32 2000) -> ()  [unwired: 1 out]
                  }
                  frame #8 {
                    n1003 = while {
                      stop <- w5037 stop-if-true
                      n1004 = local read "Raster Scanning..."() -> (w5040:bool)
                      n1005 = local read "Saving..."() -> (w5038:bool)
                      n1006 = Wait (ms)(milliseconds to wait=u32 100) -> ()  [unwired: 1 out]
                      n1007 = Not(x=w5038) -> (.not. x?=w5036:bool)
                      n1008 = Not(x=w5040) -> (.not. x?=w5039:bool)
                      n1009 = And(x=w5039, y=w5036) -> (x .and. y?=w5037:bool)
                    }
                  }
                  frame #9 {
                    n1010 = property on="Trap Delta (MHz)" class="DigNum (strict)"("Val(Sgnl)"=w5044) -> ()  [unwired: 2 in, 2 out]
                    n1011 = property on="Saved AOD Raster Scan Parameter Sets" class="Arr (strict)"("Index Values"=u32[] [0]) -> ()  [unwired: 2 in, 2 out]
                    n1012 = property on="Save ave N" class="DigNum (strict)"("Val(Sgnl)"=w5042) -> ()  [unwired: 2 in, 2 out]
                  }
                  frame #10 {
                    n1013 = Wait (ms)(milliseconds to wait=u32 500) -> ()  [unwired: 1 out]
                  }
                  frame #11 {
                    n1014 = property on="Load parameters" class="Bool (strict)"("Val(Sgnl)"=TRUE ("Value (Signaling)")) -> ()  [unwired: 2 in, 2 out]
                  }
                }
              }
            }
          }
          frame #7 {
            n1015 = property on="Read Cal" class="Bool (strict)"("Val(Sgnl)"=TRUE ("Value (Signaling)")) -> ()  [unwired: 2 in, 2 out]
          }
          frame #8 {
            n1016 = Wait (ms)(milliseconds to wait=u32 500) -> ()  [unwired: 1 out]
          }
          frame #9 {
            n1017 = property on="Fish for Tether" class="Bool (strict)"("Val(Sgnl)"=FALSE ("Value (Signaling)")) -> ()  [unwired: 2 in, 2 out]
          }
        }
      }
      event "Dump Beads": Value Change {
        # "SCRIPT TO REMOVE BOTH BEADS FROM THE TRAPS. TURNS ON LIGHT WHICH INDICATES THAT STAGE IS MOVING. THEN STOPS SAVING DATA. \nSETS Sample Channel Flow TO TRUE. STOPS INTERLACING GREEN FLUORESCENCE. TURNS OFF Tether INDICATOR BECAUSE WE ARE THROWING IT\nAWAY. SHUTS OFF TRAP POSITION FEEDBACK."
        n1018 = event-data() -> ()  [unwired: 1 in, 5 out]
        n1019 = flat-sequence {
          frame #0 {
            w5051 = FALSE ("Fl. Triggered...")
            w5052 = TRUE ("Stage Moving")
            n1020 = local read "Saving..."() -> (w5053:bool)
            n1021 = local write "Fl. Triggered..."(w5051) -> ()
            n1022 = local write "Stage Moving"(w5052) -> ()
            n1023 = local write "Tether"(w5051) -> ()
            n1024 = property on="Green Laser ON/Interlacing" class="Bool (strict)"("Val(Sgnl)"=w5051) -> ()  [unwired: 2 in, 2 out]
            n1025 = property on="Trap Pos. FB ON" class="Bool (strict)"("Val(Sgnl)"=w5051) -> ()  [unwired: 2 in, 2 out]
            n1026 = property on="Sample Channel Flow" class="Bool (strict)"("Val(Sgnl)"=w5052) -> ()  [unwired: 2 in, 2 out]
            n1027 = local write "Stop Saving"(w5053) -> ()
          }
          frame #1 {
            w5054 = FALSE ("Value (Signaling)")
            # "TURNS TRAPS OFF SO THAT\nBEADS REMAIN AT DUMP \nBEADS POSITION"
            n1028 = property on="Trap 1 (ON/OFF)" class="Bool (strict)"("Val(Sgnl)"=w5054) -> ()  [unwired: 2 in, 2 out]
            n1029 = property on="Trap 2 (ON/OFF)" class="Bool (strict)"("Val(Sgnl)"=w5054) -> ()  [unwired: 2 in, 2 out]
            n1030 = call <vilib>:"Beep.vi"() -> ()  [unwired: 3 in, 9 out]
          }
          frame #2 {
            n1031 = local read "Cal @ (MHz)"() -> (w5055:dbl)
            n1032 = property on="Trap Delta (MHz)" class="DigNum (strict)"("Val(Sgnl)"=w5055) -> ()  [unwired: 2 in, 2 out]
          }
        }
      }
      event "Dip for Protein": Value Change {
        n1033 = event-data() -> ()  [unwired: 1 in, 5 out]
        n1034 = flat-sequence {
          frame #0 {
            n1035 = case shown="True" "Move Trap Before?" {
              frame False {
              }
              frame True {
                n1036 = property on="Trap Delta (MHz)" class="DigNum (strict)"("Val(Sgnl)"="Dip Trap Delta 1 (MHz)") -> ()  [unwired: 2 in, 2 out]
              }
            }
          }
          frame #1 {
            n1037 = Multiply(x="Duration (s)", y=1000.0) -> (x*y=w5059:dbl)
            n1038 = Wait (ms)(milliseconds to wait=w5059) -> ()  [unwired: 1 out]
          }
          frame #2 {
            n1039 = case shown="True" "Move Trap After?" {
              frame False {
              }
              frame True {
                n1040 = property on="Trap Delta (MHz)" class="DigNum (strict)"("Val(Sgnl)"="Dip Trap Delta 2 (MHz)") -> ()  [unwired: 2 in, 2 out]
              }
            }
          }
          frame #3 {
            n1041 = case shown="True" "Green ON After?" {
              frame False {
              }
              frame True {
                n1042 = property on="Green Laser ON/Interlacing" class="Bool (strict)"("Val(Sgnl)"=TRUE ("Value (Signaling)")) -> ()  [unwired: 2 in, 2 out]
              }
            }
          }
          frame #4 {
            n1043 = Wait (ms)(milliseconds to wait=u32 500) -> ()  [unwired: 1 out]
          }
          frame #5 {
            n1044 = case shown="True" "Save Data After?" {
              frame False {
              }
              frame True {
                n1045 = property on="Start Saving" class="Bool (strict)"("Val(Sgnl)"=TRUE ("Value (Signaling)")) -> ()  [unwired: 2 in, 2 out]
              }
            }
          }
        }
      }
      event "Profile": Value Change {
        n1046 = event-data() -> ()  [unwired: 1 in, 5 out]
        n1047 = flat-sequence {
          frame #0 {
            w5069 = 0.0 ("element")
            n1048 = Build Array(w5069, "Y change (mm)", w5069) -> ()  [unwired: 1 out]
          }
          frame #1 {
            # "stop saving"
            n1049 = local write "Stop Saving"(TRUE ("Stop Saving")) -> ()
            n1050 = local write "Stage Moving"(FALSE ("Stage Moving")) -> ()
          }
        }
      }
      event "Got ADig bead": Value Change {
        n1051 = event-data() -> ()  [unwired: 1 in, 5 out]
        n1052 = property on="Move Cap. 1 (DNA Top)" class="Bool (strict)"("Val(Sgnl)"=TRUE ("Value (Signaling)")) -> ()  [unwired: 2 in, 2 out]
        n1053 = property on="Inject Bottom" class="Bool (strict)"("Val(Sgnl)"=FALSE ("Value (Signaling)")) -> ()  [unwired: 2 in, 2 out]
      }
      event "Got DNA bead": Value Change {
        n1054 = event-data() -> ()  [unwired: 1 in, 5 out]
        n1055 = property on="Cal/Data Acq. Spot" class="Bool (strict)"("Val(Sgnl)"=TRUE ("Value (Signaling)")) -> ()  [unwired: 2 in, 2 out]
        n1056 = property on="Inject Top" class="Bool (strict)"("Val(Sgnl)"=FALSE ("Value (Signaling)")) -> ()  [unwired: 2 in, 2 out]
      }
      event "Take Stepping Data": Value Change {
        n1057 = event-data() -> ()  [unwired: 1 in, 5 out]
        n1058 = local read "Save ave N"() -> (w5087:dbl)
        n1059 = flat-sequence {
          tunnel: w5087 -> [w5089]
          tunnel: [w5089] -> w5082
          tunnel: [w5091] -> w5083
          tunnel: w5082 -> [w5091]
          tunnel: [w5093] -> w5084
          tunnel: w5083 -> [w5093]
          tunnel: [w5096] -> w5085
          tunnel: w5084 -> [w5096]
          tunnel: [w5098] -> w5086
          tunnel: w5085 -> [w5098]
          tunnel: [w5100] -> w5080
          tunnel: w5086 -> [w5100]
          tunnel: w5080 -> [w5103]
          tunnel: [w5103] -> w5079
          tunnel: w5079 -> [w5104]
          tunnel: [w5104] -> w5081
          tunnel: w5081 -> [w5110]
          frame #0 {
            n1060 = property on="Save ave N" class="DigNum (strict)"("Val(Sgnl)"="Save ave factor") -> ()  [unwired: 2 in, 2 out]
          }
          frame #1 {
            n1061 = Wait (ms)(milliseconds to wait=u32 100) -> ()  [unwired: 1 out]
          }
          frame #2 {
            n1062 = local read "Offset 2 Start (MHz)"() -> (w5095:dbl)
            n1063 = property on="Saved AOD Raster Scan Parameter Sets" class="Arr (strict)"("Index Values"=u32[] [2]) -> ()  [unwired: 2 in, 2 out]
            n1064 = property on="Trap Delta (MHz)" class="DigNum (strict)"("Val(Sgnl)"=w5095) -> ()  [unwired: 2 in, 2 out]
          }
          frame #3 {
            n1065 = property on="Load parameters" class="Bool (strict)"("Val(Sgnl)"=TRUE ("Value (Signaling)")) -> ()  [unwired: 2 in, 2 out]
          }
          frame #4 {
            n1066 = Wait (ms)(milliseconds to wait=u32 100) -> ()  [unwired: 1 out]
          }
          frame #5 {
            n1067 = property on="Trap Raster Scan" class="Bool (strict)"("Val(Sgnl)"=TRUE ("Value (Signaling)")) -> ()  [unwired: 2 in, 2 out]
          }
          frame #6 {
            n1068 = Wait (ms)(milliseconds to wait=u32 1000) -> ()  [unwired: 1 out]
          }
          frame #7 {
            n1069 = while {
              stop <- w5107 stop-if-true
              n1070 = local read "Raster Scanning..."() -> (w5109:bool)
              n1071 = local read "Saving..."() -> (w5108:bool)
              n1072 = Not(x=w5108) -> (.not. x?=w5105:bool)
              n1073 = Not(x=w5109) -> (.not. x?=w5106:bool)
              n1074 = And(x=w5106, y=w5105) -> (x .and. y?=w5107:bool)
            }
          }
          frame #8 {
            n1075 = property on="Save ave N" class="DigNum (strict)"("Val(Sgnl)"=w5110) -> ()  [unwired: 2 in, 2 out]
          }
        }
      }
      event "Step Size (nm)": Value Change {
        n1076 = event-data() -> ()  [unwired: 1 in, 5 out]
        n1077 = flat-sequence {
          frame #0 {
            n1078 = property on="Saved AOD Raster Scan Parameter Sets" class="Arr (strict)"("Index Values"=u32[] [1]) -> ()  [unwired: 2 in, 2 out]
          }
          frame #1 {
            n1079 = Multiply(x="N Steps", y="Step Size (nm)") -> (x*y=w5112:dbl)
            n1080 = property on="Scan Speed AOD (nm/s) 2" class="DigNum (strict)"("Value"="Step Size (nm)") -> ()  [unwired: 2 in, 2 out]
            n1081 = property on="Step Size AOD (nm) 2" class="DigNum (strict)"("Value"="Step Size (nm)") -> ()  [unwired: 2 in, 2 out]
            n1082 = property on="Scan Range AOD (nm) 2" class="DigNum (strict)"("Value"=w5112) -> ()  [unwired: 2 in, 2 out]
          }
        }
      }
      event "Take Detection Laser\nImage": Value Change {
        n1083 = event-data() -> ()  [unwired: 1 in, 5 out]
        n1084 = flat-sequence {
          tunnel: [w5140] -> w5130
          tunnel: [w5139] -> w5123
          tunnel: [w5138] -> w5115
          tunnel: [w5143] -> w5131
          tunnel: w5130 -> [w5143]
          tunnel: [w5142] -> w5124
          tunnel: w5123 -> [w5142]
          tunnel: [w5141] -> w5116
          tunnel: w5115 -> [w5141]
          tunnel: [w5147] -> w5132
          tunnel: w5131 -> [w5147]
          tunnel: [w5146] -> w5125
          tunnel: w5124 -> [w5146]
          tunnel: [w5145] -> w5117
          tunnel: w5116 -> [w5145]
          tunnel: [w5153] -> w5133
          tunnel: w5132 -> [w5153]
          tunnel: [w5152] -> w5126
          tunnel: w5125 -> [w5152]
          tunnel: [w5151] -> w5118
          tunnel: w5117 -> [w5151]
          tunnel: [w5157] -> w5134
          tunnel: w5133 -> [w5157]
          tunnel: [w5156] -> w5127
          tunnel: w5126 -> [w5156]
          tunnel: [w5155] -> w5119
          tunnel: w5118 -> [w5155]
          tunnel: [w5161] -> w5135
          tunnel: w5134 -> [w5161]
          tunnel: [w5160] -> w5128
          tunnel: w5127 -> [w5160]
          tunnel: [w5159] -> w5120
          tunnel: w5119 -> [w5159]
          tunnel: [w5165] -> w5136
          tunnel: w5135 -> [w5165]
          tunnel: [w5164] -> w5129
          tunnel: w5128 -> [w5164]
          tunnel: [w5163] -> w5121
          tunnel: w5120 -> [w5163]
          tunnel: w5136 -> [w5171]
          tunnel: w5129 -> [w5170]
          tunnel: [w5168] -> w5122
          tunnel: w5121 -> [w5168]
          tunnel: w5122 -> [w5172]
          frame #0 {
            n1085 = local read "Green Laser ON/Interlacing"() -> (w5140:bool)
            n1086 = local read "Green laser mode"() -> (w5139:enum32{"Laser ON", "Laser OFF", "Interlace"})
            n1087 = local read "Green FB On/Off"() -> (w5138:bool)
          }
          frame #1 {
            n1088 = property on="Green FB On/Off" class="Bool (strict)"("Val(Sgnl)"=FALSE ("Value (Signaling)")) -> ()  [unwired: 2 in, 2 out]